vi "checkCalibStageAndCamera.vi"() -> ()   [LabVIEW 2016] (continued)
  in  "Line Coordinates":i32[](array[numeric])=[0, 1050, 2592, 1050]
  out "Matches (pixel)":T3(array[cluster]) {"Bounding Box"."y" format="%.2f"; "Bounding Box"."x" format="%.2f"; "Score" format="%.2f"; "Scale" format="%.2f"; "Angle" format="%.2f"; "Position"."y" format="%.2f"; "Position"."x" format="%.2f"}
  in  "Match parameters":T4={"Number of Matches Requested"=1, "Minimum Match Score"=600.0, "Angle Ranges"=[]}
  in  "Template File Path":path=path "E:/XYZstage+Camera_CollectedImages/12-15-2016/smallPin_sub2_12-15-2016-Gain14p44.png"
  in  "Axes Speeds [mm/s]":T5={"X Speed"=25.0, "Y Speed"=12.5, "Z Speed"=10.0}
  in  "Send stage to XYZ [mm]":T6
  in  "Move stage":bool
  in  "Home stage":bool
  out "N moves":i32=1
  out "Intensity Histogram":T7(graph)={"Starting Value"=0.0, "Incremental Value"=1.0, "Histogram"=[104, 591, 3049, 13441, 52430, 123784, 258512, 486314, 592841, 462464, 767569, 680654, 540708, 425015, 275408, 163786, 100082, 49501, 22916, 11426, 4804, 1945, 895, 353, 151, 60, 24, 10, 6, 2, 0, 1, 0, 0, 0, 0, 0, 0, 0, 0, 0, 0, 0, 0, 0, 0, 0, 0, 0, 0, 0, 0, 0, 0, 0, 0, 0, 0, 0, 0, 0, 0, 0, 0, 0, 0, 0, 0, 0, 0, 0, 0, 0, 0, 0, 0, 0, 0, 0, 0, 0, 0, 0, 0, 0, 0, 0, 0, 0, 0, 0, 0, 0, 0, 0, 0, 0, 0, 0, 0, 0, 0, 0, 0, 0, 1, 0, 0, 0, 0, 0, 0, 0, 0, 0, 0, 0, 0, 0, 0, 0, 0, 0, 0, 0, 0, 0, 0, 0, 0, 0, 0, 0, 0, 0, 0, 0, 0, 0, 0, 0, 0, 0, 0, 0, 1, 0, 0, 0, 0, 0, 0, 0, 0, 0, 0, 0, 0, 0, 0, 0, 0, 0, 0, 0, 0, 0, 0, 0, 0, 0, 0, 0, 0, 0, 0, 0, 0, 0, 0, 0, 0, 0, 0, 0, 0, 0, 0, 0, 0, 0, 0, 0, 0, 0, 0, 0, 0, 0, 0, 0, 0, 0, 0, 0, 0, 0, 0, 0, 0, 0, 0, 0, 0, 0, 0, 0, 0, 0, 0, 0, 0, 0, 0, 0, 0, 0, 0, 0, 0, 0, 0, 0, 0, 0, 0, 0, 0, 0, 0, 0, 0, 0, 0, 0, 0, 0, 0, 0, 0, 0, 0, 0, 0, 0, 0]}
  out "Moving":bool
  out "Homed":bool
  in  "Stop Program":bool
  out "XYZ Stage Current Position":T8={"X [-750, 750 mm]"=0.008702056884765625, "Y [-150, 30 mm]"=-0.004916462646484375, "Z [-50, 50 mm]"=0.0046}
  out "Error report":errorcluster
  out "Image":T9(plugin-control) caption="Image Out"
  in  "Camera Name":refnum<k21>="cam0" caption="IMAQdx Session"
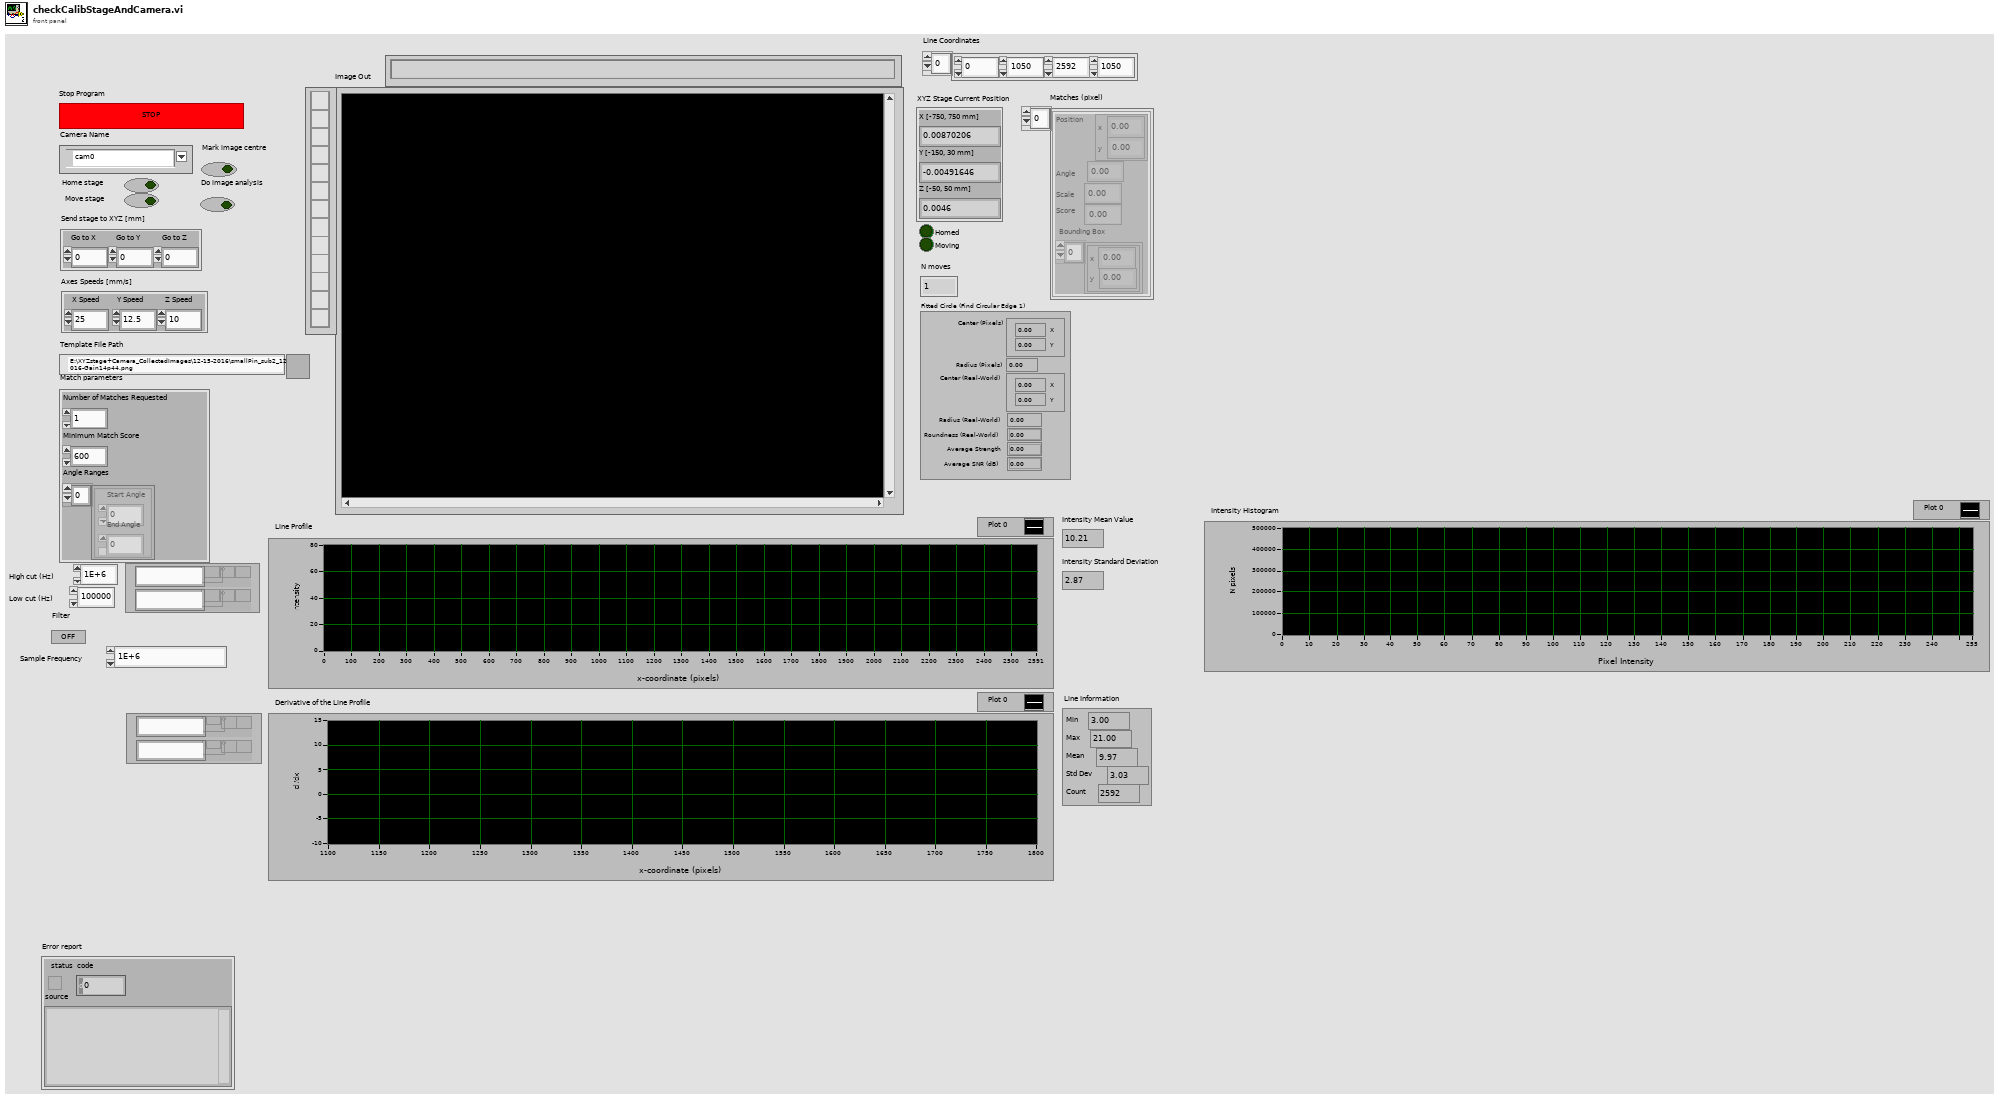
[diagram p1: front panel]
types:
  T1 = cluster{"Center (Pixels)":cluster{"X":sgl, "Y":sgl}, "Radius (Pixels)":dbl, "Center (Real-World)":cluster{"X":sgl, "Y":sgl}, "Radius (Real-World)":dbl, "Roundness (Real-World)":dbl, "Average Strength":dbl, "Average SNR (dB)":dbl}
  T2 = cluster{"Min":sgl, "Max":sgl, "Mean":sgl, "Std Dev":sgl, "Count":i32}
  T3 = cluster{"Position":cluster{"x":sgl, "y":sgl}, "Angle":sgl, "Scale":sgl, "Score":sgl, "Bounding Box":cluster{"x":sgl, "y":sgl}[]}[]
  T4 = cluster{"Number of Matches Requested":i32, "Minimum Match Score":sgl, "Angle Ranges":cluster{"Start Angle":sgl, "End Angle":sgl}[]}
  T5 = cluster{"X Speed":dbl, "Y Speed":dbl, "Z Speed":dbl}
  T6 = cluster{"Go to X":dbl, "Go to Y":dbl, "Go to Z":dbl}
  T7 = cluster{"Starting Value":sgl, "Incremental Value":sgl, "Histogram":u32[]}
  T8 = cluster{"X [-750, 750 mm]":dbl, "Y [-150, 30 mm]":dbl, "Z [-50, 50 mm]":dbl}
  T9 = typedef "IMAQ Image.ctl" = refnum<image>
  T10 = typedef "Image Type" = u32
  T11 = typedef "IMAQdx.ctl" = refnum<k21>
  T12 = cluster{"X Position Feedback":dbl, "Y Position Feedback":dbl, "Z Position Feedback":dbl}
  T13 = typedef "NI_AALBase.lvlib/Filter Passband Type.ctl" = enum32{"Lowpass", "Highpass", "Bandpass", "Bandstop"}
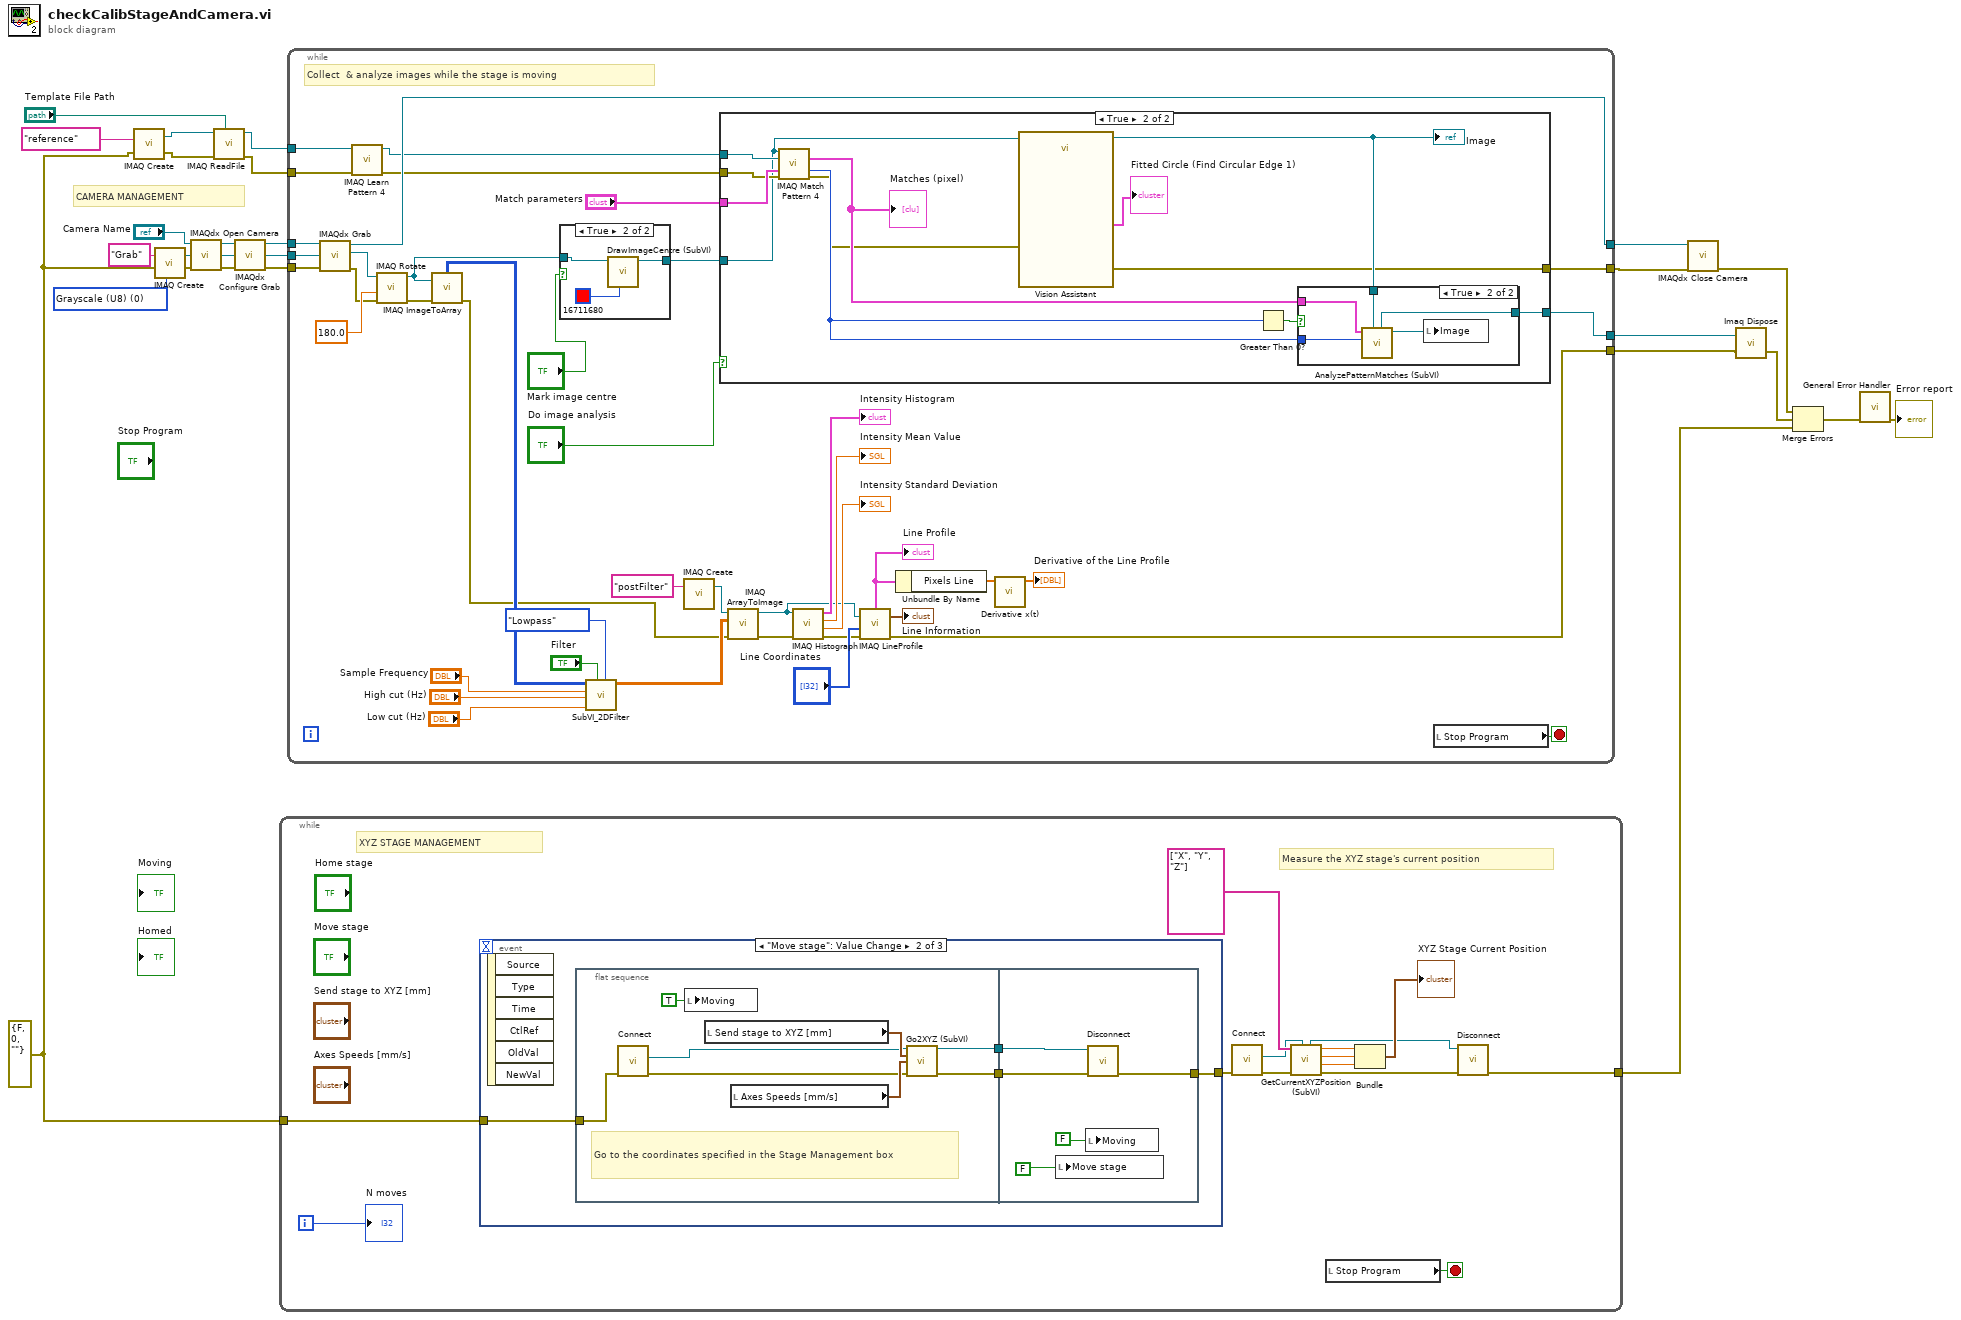
[diagram p0: block diagram]
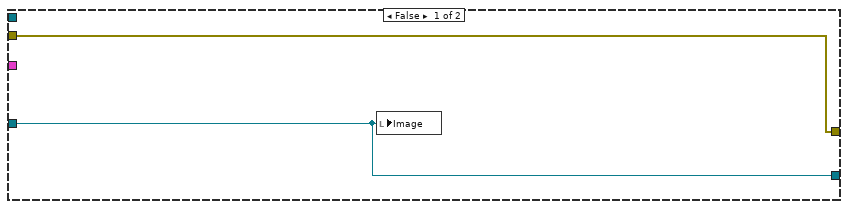
[diagram p2: hidden frame]
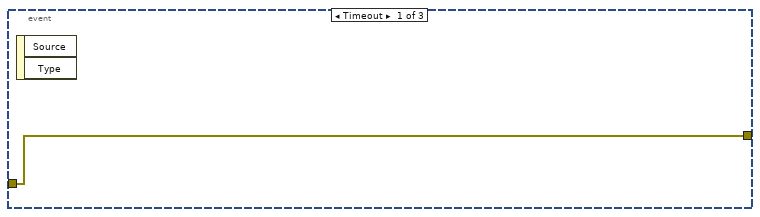
[diagram p5: hidden frame]
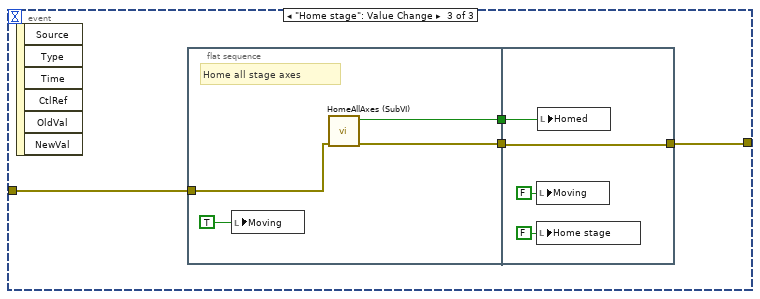
[diagram p6: hidden frame]
diagram:
  w20 = T10 0 items=["Grayscale (U8)", "Grayscale (I16)", "Grayscale (SGL)", "Complex (CSG)", "RGB (U32)", "HSL (U32)", "RGB (U64)", "Grayscale (U16)"] ("Image Type")
  w4 = errorcluster {"status"=FALSE, "code"=0, "source"=""} ("error in (no error)")
  # "CAMERA MANAGEMENT"
  n1 = call "IMAQ Create"("Image Name"="reference", "error in (no error)"=w4) -> ("New Image"=w10:T9, "error out"=w9:errorcluster)  [unwired: 3 in]
  n2 = call "IMAQ Create"("Image Name"="Grab", "Image Type"=w20, "error in (no error)"=w4) -> ("New Image"=w16:T9, "error out"=w25:errorcluster)  [unwired: 1 in, 1 out]
  n3 = call <vilib>:"IMAQdx Open Camera.vi"("error in"=w25, "Session In"="Camera Name") -> ("error out"=w22:errorcluster, "Session Out"=w23:T11)  [unwired: 1 in, 7 out]
  n4 = call "IMAQ ReadFile"("File Path"="Template File Path", "error in (no error)"=w9, "Image"=w10) -> ("error out"=w6:errorcluster, "Image Out"=w7:T9)  [unwired: 4 in, 3 out]
  n5 = call <vilib>:"IMAQdx Configure Grab.vi"("error in"=w22, "Session In"=w23) -> ("error out"=w17:errorcluster, "Session Out"=w18:T11)  [unwired: 8 out]
  n6 = while {
    tunnel: w4 -> [w30]
    tunnel: [w31] -> w13
    i -> [w34]
    stop <- w32 stop-if-true
    # "XYZ STAGE MANAGEMENT"
    # "Measure the XYZ stage's current position"
    n7 = event shown="[1] \"Move stage\": Value Change" {
      selector: _ -> [_ _ _]
      dyn-events: _ -> [_ _ _]
      timeout: _ -> [_ _ _]
      tunnel: [w40 w41 w60] -> w27
      tunnel: w30 -> [w40 w42 w58]
      event Timeout {
        n8 = event-data() -> ()  [unwired: 1 in, 2 out]
      }
      event "Move stage": Value Change {
        n9 = event-data() -> ()  [unwired: 1 in, 6 out]
        n10 = flat-sequence {
          tunnel: [w52] -> w44
          tunnel: [w51] -> w43
          tunnel: w42 -> [w45]
          tunnel: w44 -> [w55]
          tunnel: w43 -> [w54]
          tunnel: [w53] -> w41
          frame #0 {
            # "Go to the coordinates specified in the Stage Management box"
            n11 = call "Connect.vi"("error in (no error)"=w45) -> ("error out"=w47:errorcluster, "controller"=w46:refnum<k24>)  [unwired: 9 in]
            n12 = local write "Moving"(TRUE ("Moving")) -> ()
            n13 = local read "Send stage to XYZ [mm]"() -> (w49:T6)
            n14 = local read "Axes Speeds [mm/s]"() -> (w48:T5)
            n15 = call "Go2XYZ (SubVI).vi"(".NET Refnum in"=w46, "Go to Coordinates"=w49, "Axis Speeds"=w48, "error in (no error)"=w47) -> (".NET Refnum out"=w52:refnum<k24>, "error out"=w51:errorcluster)  [unwired: 8 in, 2 out]
          }
          frame #1 {
            n16 = local write "Move stage"(FALSE ("Move stage")) -> ()
            n17 = local write "Moving"(FALSE ("Moving")) -> ()
            n18 = call "Disconnect.vi"("error in (no error)"=w54, "controller"=w55) -> ("error out"=w53:errorcluster)  [unwired: 9 in]
          }
        }
      }
      event "Home stage": Value Change {
        n19 = event-data() -> ()  [unwired: 1 in, 6 out]
        n20 = flat-sequence {
          tunnel: [w64] -> w61
          tunnel: [w63] -> w59
          tunnel: w58 -> [w62]
          tunnel: w61 -> [w67]
          tunnel: [w66] -> w60
          tunnel: w59 -> [w66]
          frame #0 {
            # "Home all stage axes"
            n21 = local write "Moving"(TRUE ("Moving")) -> ()
            n22 = call "HomeAllAxes (SubVI).vi"("error in (no error)"=w62) -> ("error out"=w63:errorcluster, "completed"=w64:bool)  [unwired: 8 in, 1 out]
          }
          frame #1 {
            n23 = local write "Moving"(FALSE ("Moving")) -> ()
            n24 = local write "Home stage"(FALSE ("Home stage")) -> ()
            n25 = local write "Homed"(w67) -> ()
          }
        }
      }
    }
    n26 = call "Connect.vi"("error in (no error)"=w27) -> ("error out"=w29:errorcluster, "controller"=w28:refnum<k24>)  [unwired: 9 in]
    n27 = call "GetCurrentXYZPosition (SubVI).vi"(".NET Refnum in - Device"=w28, "error in (no error)"=w29, "Axes Names"=string[] ["X", "Y", "Z"]) -> ("error out"=w33:errorcluster, "Z Position Feedback"=w39:dbl, "Y Position Feedback"=w38:dbl, "X Position Feedback"=w37:dbl, ".NET Refnum out  - Device"=w26:refnum<k24>)  [unwired: 3 in]
    n28 = local read "Stop Program"() -> (w32:bool)
    n29 = Bundle("X Position Feedback"=w37, "Y Position Feedback"=w38, "Z Position Feedback"=w39) -> (→"XYZ Stage Current Position":T12)  [unwired: 1 in]
    n30 = call "Disconnect.vi"("error in (no error)"=w33, "controller"=w26) -> ("error out"=w31:errorcluster)  [unwired: 9 in]
    "N moves" <- w34
  }
  n31 = while {
    tunnel: w18 -> [w110]
    tunnel: w17 -> [w109]
    tunnel: w16 -> [w108]
    tunnel: [w107] -> w15
    tunnel: [w94] -> w3
    tunnel: w7 -> [w105]
    tunnel: w6 -> [w104]
    tunnel: [w80] -> w5
    tunnel: [w74] -> w1
    stop <- w111 stop-if-true
    # "Collect  & analyze images while the stage is moving"
    n32 = call <vilib>:"IMAQdx Grab.vi"("error in"=w109, "Image In"=w108, "Session In"=w110) -> ("error out"=w78:errorcluster, "Image Out"=w100:T9, "Session Out"=w107:T11)  [unwired: 1 in, 5 out]
    n33 = call "IMAQ Learn Pattern 4"("error in (no error)"=w104, "Image"=w105) -> ("error out"=w101:errorcluster, "Template Image Out"=w103:T9)  [unwired: 7 in, 1 out]
    n34 = call "IMAQ Rotate"("error in (no error)"=w78, "Angle (degrees)"=sgl 180.0, "Image Src"=w100) -> ("error out"=w77:errorcluster, "Image Dst Out"=w73:T9)  [unwired: 7 in]
    n35 = call "IMAQ ImageToArray"("error in (no error)"=w77, "Image"=w73) -> ("error out"=w75:errorcluster, "Image Pixels (U8)"=w83:u8[][])  [unwired: 2 in, 3 out]
    n36 = case shown="True" "Mark image centre" {
      tunnel: w73 -> [w132 w135]
      tunnel: [w132 w134] -> w72
      frame False {
      }
      frame True {
        n37 = call "DrawImageCentre (SubVI).vi"("Axis colour"=u32 16711680, "Refnum in"=w135) -> ("Refnum out"=w134:T9)  [unwired: 8 in, 1 out]
      }
    }
    n38 = call "SubVI_2DFilter.vi"("Input"=w83, "Sample Frequency"="Sample Frequency", "High cut (Hz)"="High cut (Hz)", "Low cut (Hz)"="Low cut (Hz)", "Filter"="Filter", "Filter type"=Filter_Passband_Type."Lowpass") -> ("Filter output"=w89:dbl[][])  [unwired: 4 in]
    n39 = call "IMAQ Create"("Image Name"="postFilter") -> ("New Image"=w87:T9)  [unwired: 4 in, 1 out]
    n40 = case shown="True" "Do image analysis" {
      tunnel: w103 -> [_ w125]
      tunnel: "Match parameters" -> [_ w124]
      tunnel: w101 -> [w112 w123]
      tunnel: [w113 w117] -> w80
      tunnel: [w112 w115] -> w74
      tunnel: w72 -> [w113 w114]
      frame False {
        n41 = local write "Image"(w113) -> ()
      }
      frame True {
        n42 = call "IMAQ Match Pattern 4"("Image"=w114, "Template Image"=w125, "Parameters"=w124, "error in (no error)"=w123) -> ("Matches (pixel)"=w121:T3, "Number of Matches"=w120:i32, "error out"=w116:errorcluster)  [unwired: 7 in, 2 out]
        "Matches (pixel)" <- w121
        n43 = call "Vision Assistant"("Image In"=w114, "error in"=w116) -> ("Image Out"=w118:T9, "Fitted Circle (Find Circular Edge 1)"=→"Fitted Circle (Find Circular Edge 1)":T1, "error out"=w115:errorcluster)  [unwired: 23 in]
        "Image" <- w118
        n44 = Greater Than 0?(x=w120) -> (x > 0?=w122:bool)
        n45 = case shown="True" w122 {
          tunnel: w120 -> [_ w131]
          tunnel: w121 -> [_ w130]
          tunnel: w118 -> [w126 w128]
          tunnel: [w126 w127] -> w117
          frame False {
          }
          frame True {
            n46 = call "AnalyzePatternMatches (SubVI).vi"("Image in"=w128, "Number of Matches"=w131, "Matches (pixel)"=w130) -> ("Display with box"=w129:T9, "Image out"=w127:T9)  [unwired: 5 in, 2 out]
            n47 = local write "Image"(w129) -> ()
          }
        }
      }
    }
    n48 = call "IMAQ ArrayToImage"("error in (no error)"=w75, "Image Pixels (U8)"=w89, "Image"=w87) -> ("error out"=w79:errorcluster, "Image Out"=w86:T9)  [unwired: 7 in]
    n49 = call "IMAQ Histograph"("error in (no error)"=w79, "Image"=w86) -> ("error out"=w95:errorcluster, "Standard  Deviation"=→"Intensity Standard Deviation":sgl, "Mean Value"=→"Intensity Mean Value":sgl, "Histogram Graph"=→"Intensity Histogram":T7)  [unwired: 6 in]
    n50 = call "IMAQ LineProfile"("error in (no error)"=w95, "Line Coordinates"="Line Coordinates", "Image"=w86) -> ("error out"=w94:errorcluster, "Line Graph"=w93:cluster{"x0":sgl, "dx":sgl, "Pixels Line":sgl[]}, "Line Information"=→"Line Information":T2)  [unwired: 2 in, 1 out]
    "Line Profile" <- w93
    n51 = Unbundle By Name(w93) -> ("Pixels Line"=w92:sgl[])
    n52 = call <vilib>:"Derivative x(t).vi"("X"=w92) -> ("dX/dt"=→"Derivative of the Line Profile":dbl[])  [unwired: 9 in, 1 out]
    n53 = local read "Stop Program"() -> (w111:bool)
  }
  n54 = call <vilib>:"IMAQdx Close Camera.vi"("error in"=w1, "Session In"=w15) -> ("error out"=w2:errorcluster)  [unwired: 9 out]
  n55 = call "Imaq Dispose"("Image"=w5, "error in (no error)"=w3) -> ("error out"=w14:errorcluster)  [unwired: 4 in]
  n56 = Merge Errors(w2, w14, w13) -> (w12:errorcluster)
  n57 = call <vilib>:"General Error Handler.vi"("error in (no error)"=w12) -> ("error out"=→"Error report":errorcluster)  [unwired: 2 in, 12 out]
